vi "IV_ZAL_2015640414_P5.vi"(7 "Enum":T2(ring), 8 "error in":errorcluster, 10 "OPERADORES":T1={"Desplazamiento X"=0.0, "Desplazamiento Y"=500.0, "Giro"=0.0, "ZOOM"=0.0} {"ZOOM" min=0.1 max=10.0 step=0.01 scale=0.1..3.7; "Giro" scale=-360.0..360.0; "Desplazamiento Y" min=-500.0 max=500.0 step=1.0 scale=-200.0..200.0; "Desplazamiento X" min=-500.0 max=500.0 step=1.0 scale=-200.0..200.0}, 11 "IMAGEN 1":path) -> (0 "error out":errorcluster, 1 "HISTOGRAMA":dbl[][](graph), 2 "IMAGEN MODIFICADA":picture, 3 "IMAGEN ORIGINAL":picture)   [LabVIEW 2016]
doc: "SubVI para poder realizar distintas operaciones entre imagenes."
uses:
  <vilib>/imath/engines/lvmath2/RunTimeEngine/BuiltInFunctions/round/NIMS_round(DBL-S).vi
  <vilib>/imath/engines/lvmath2/RunTimeEngine/NodeEndStatement/NIMS_NodeEndStatement_Output.vi
  <instcachedir>/0/NIMS_NodeEndStatement_Output_53EC0D466D134D7ABD903AC30B43404B.lvgen/NIMS_NodeEndStatement_Output_53EC0D466D134D7ABD903AC30B43404B_010.vi
  <vilib>/imath/engines/lvmath2/RunTimeEngine/ErrorHandling/NIMS_Finalize Error.vi
  <instcachedir>/0/NIMS_NodeEndStatement_Output_53EC0D466D134D7ABD903AC30B43404B.lvgen/NIMS_NodeEndStatement_Output_53EC0D466D134D7ABD903AC30B43404B_001.vi
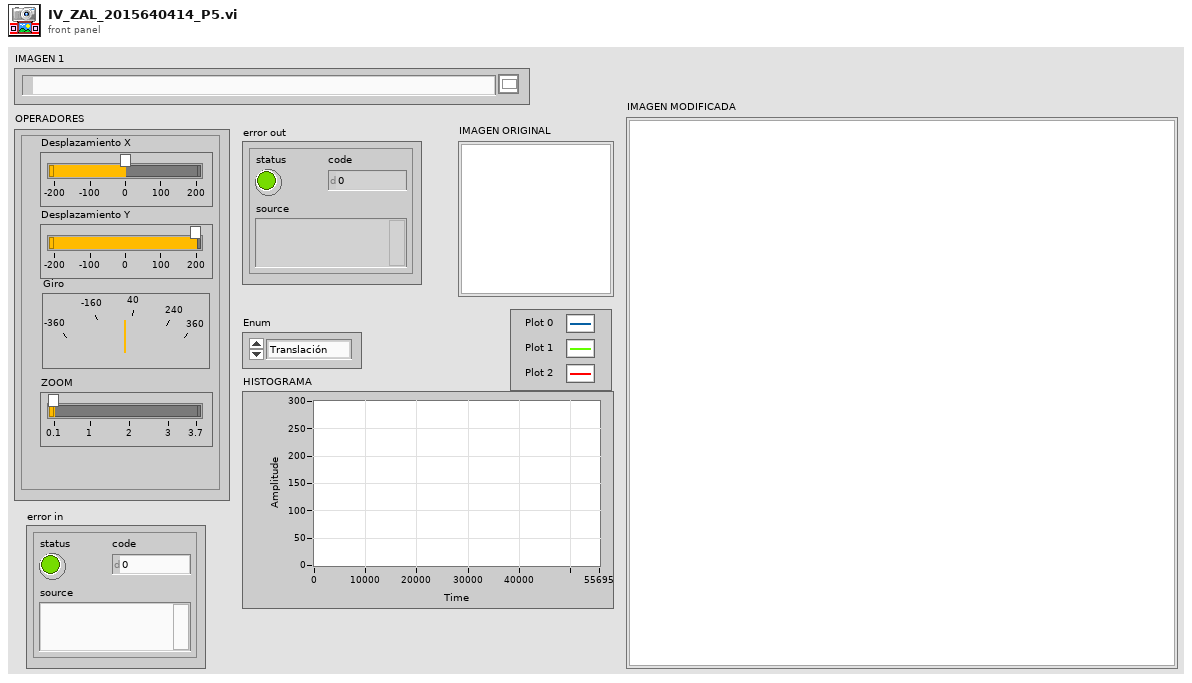
[diagram p1: front panel]
types:
  T1 = cluster{"Desplazamiento X":dbl, "Desplazamiento Y":dbl, "Giro":dbl, "ZOOM":dbl}
  T2 = enum16{"Translación", "Rotación", "Zoom", "GIROH", "GIROV", "Extracción", "Sustitución", "UNION"}
  T3 = typedef "imagedata.ctl" = cluster{"image type":i32, "image depth":i32, "image":u8[], "mask":u8[], "colors":u32[], "Rectangle":cluster{"left":i16, "top":i16, "right":i16, "bottom":i16}}
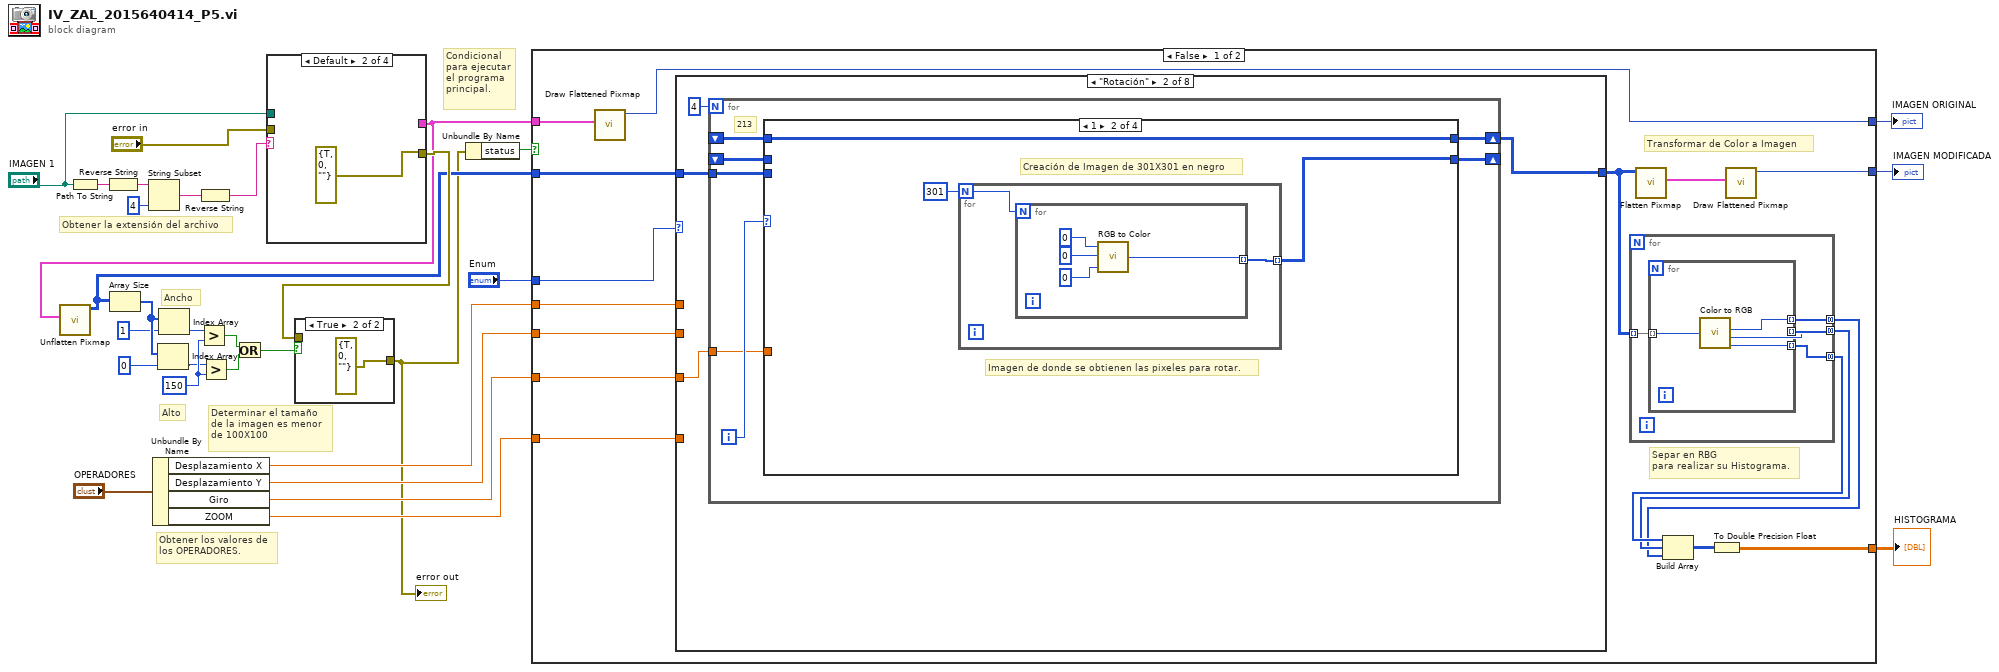
[diagram p0: block diagram]
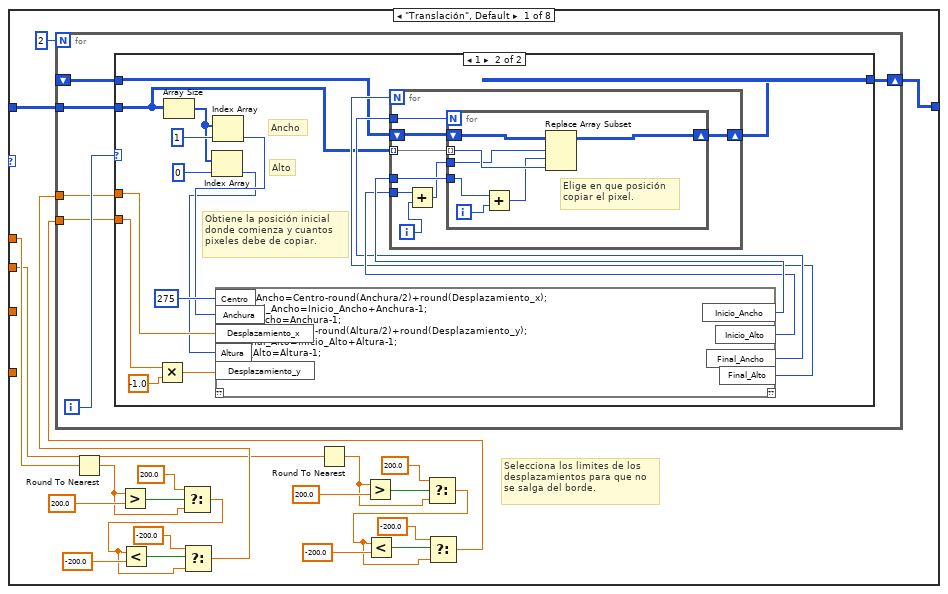
[diagram p3: hidden frame]
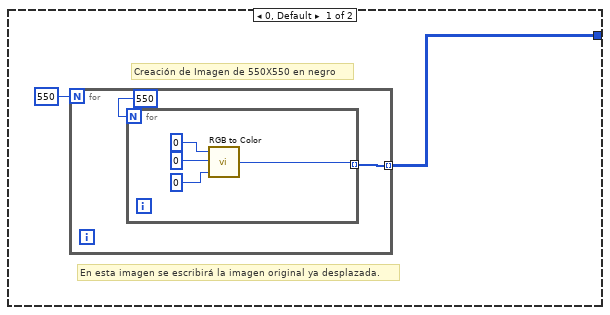
[diagram p4: hidden frame]
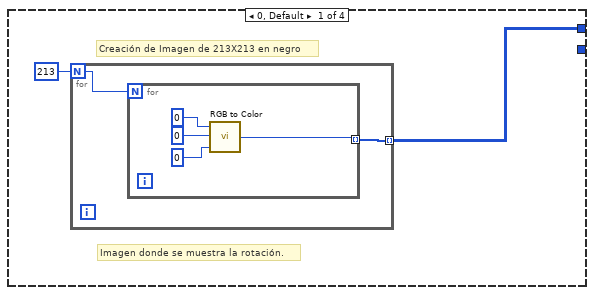
[diagram p5: hidden frame]
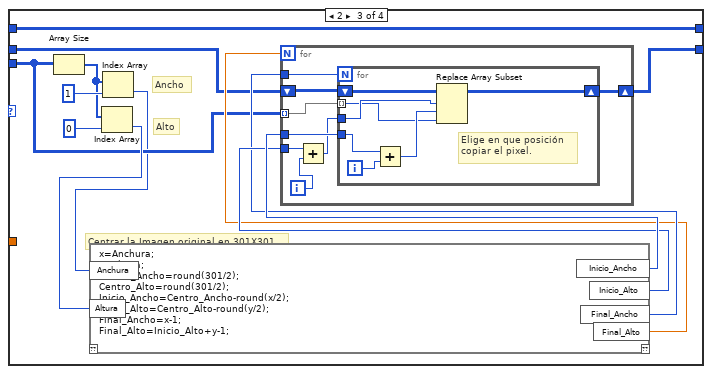
[diagram p6: hidden frame]
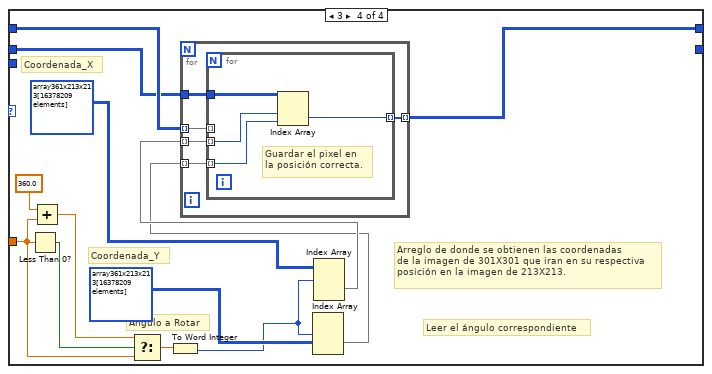
[diagram p7: hidden frame]
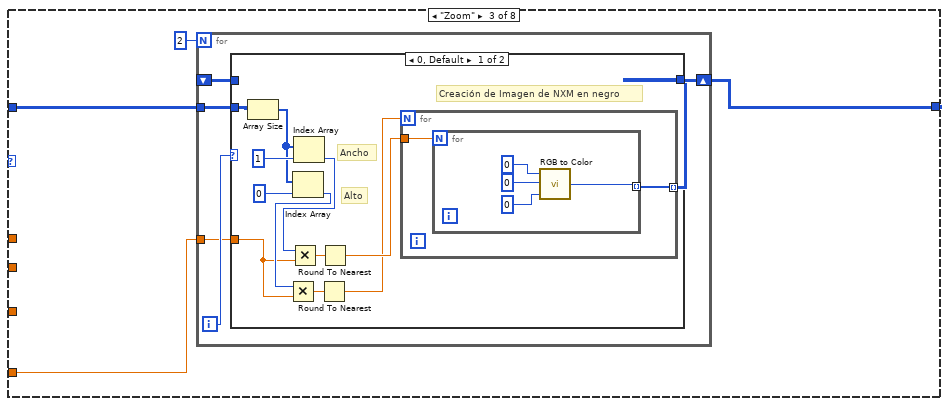
[diagram p8: hidden frame]
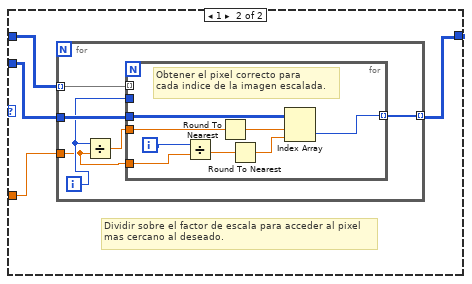
[diagram p9: hidden frame]
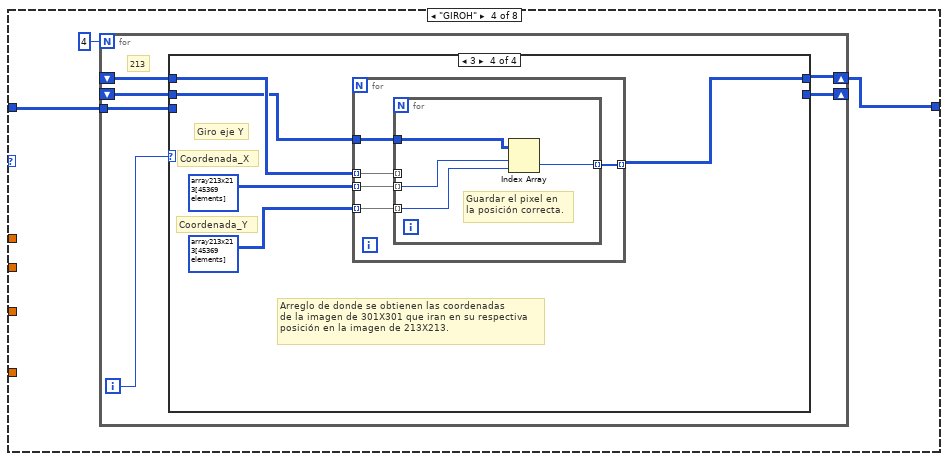
[diagram p10: hidden frame]
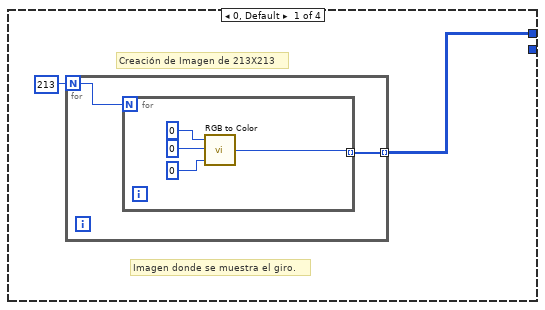
[diagram p11: hidden frame]
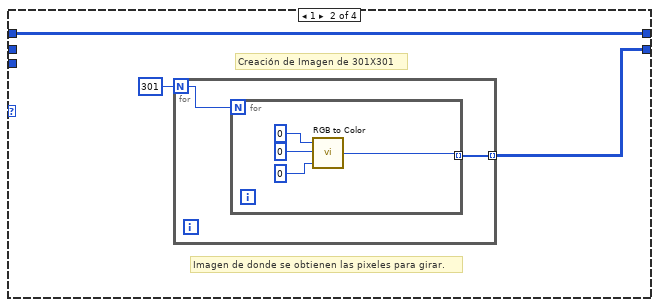
[diagram p12: hidden frame]
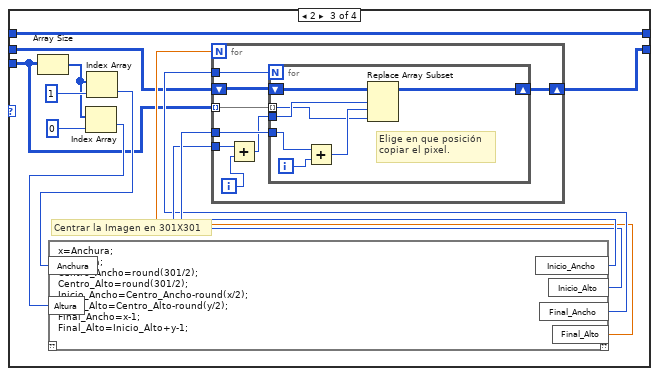
[diagram p13: hidden frame]
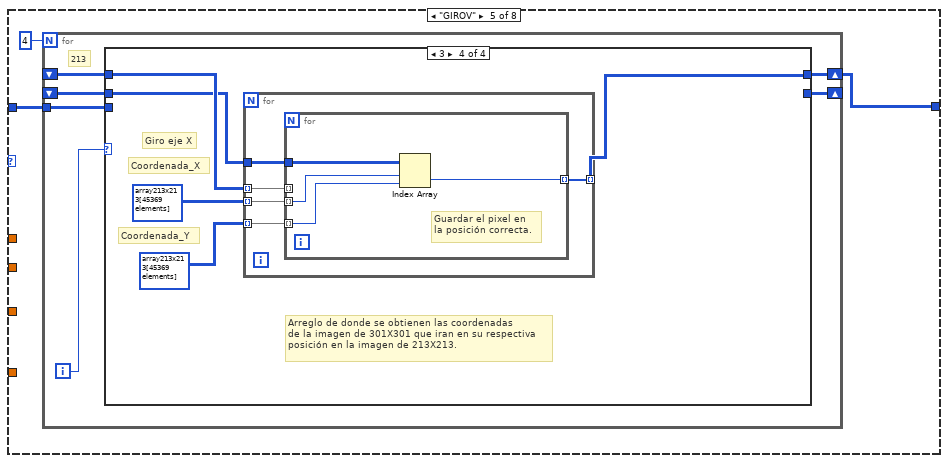
[diagram p14: hidden frame]
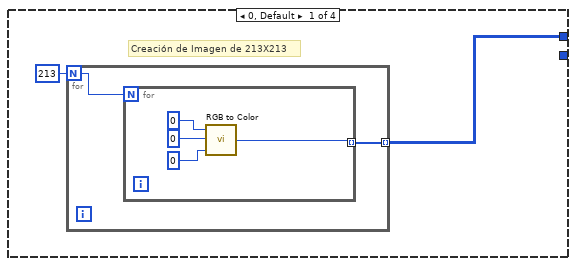
[diagram p15: hidden frame]
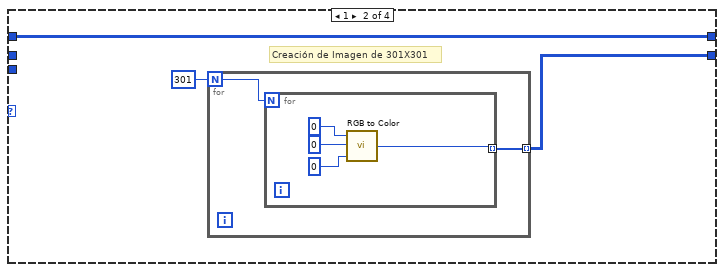
[diagram p16: hidden frame]
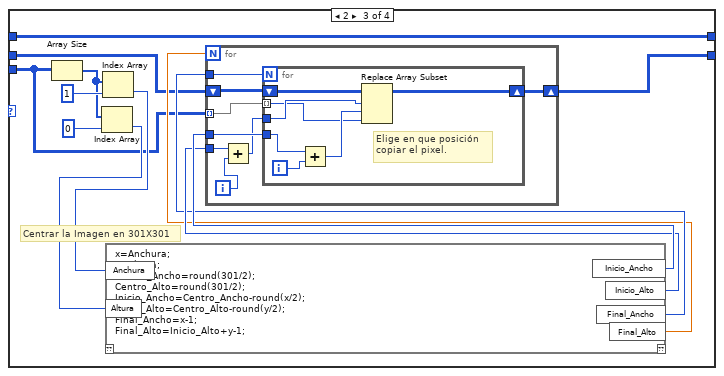
[diagram p17: hidden frame]
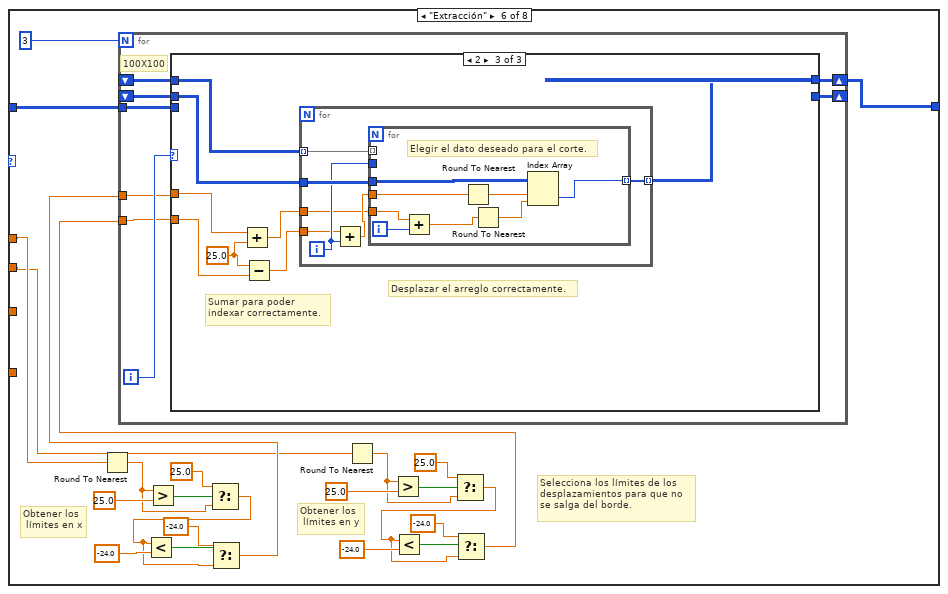
[diagram p18: hidden frame]
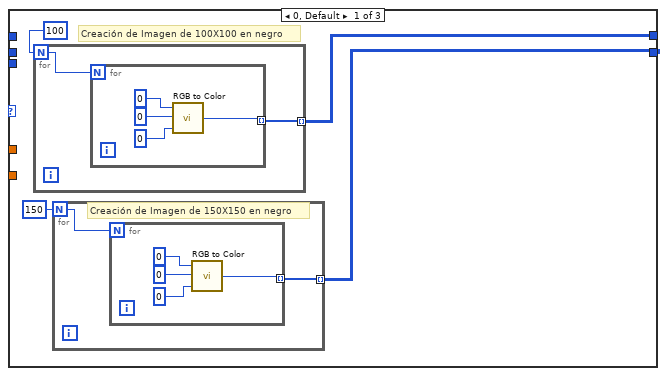
[diagram p19: hidden frame]
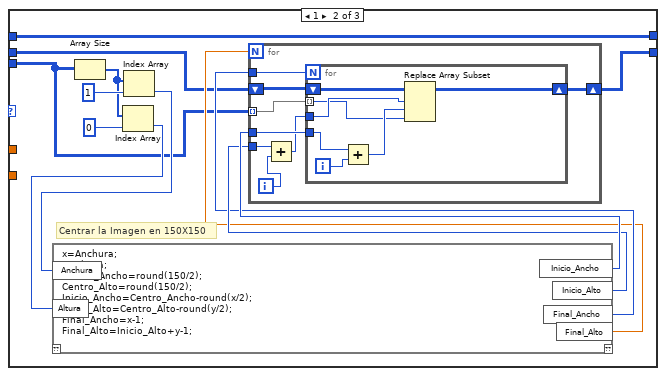
[diagram p20: hidden frame]
diagram:
  w18 = 150 ("y")
  # "Condicional\npara ejecutar\nel programa\nprincipal."
  # "Obtener los valores de\nlos OPERADORES."
  # "Determinar el tamaño\nde la imagen es menor\nde 100X100"
  # "Obtener la extensión del archivo"
  # "Alto"
  # "Ancho"
  n1 = Path To String(path="IMAGEN 1") -> (string=w1:string)
  n2 = Reverse String(1:w1) -> (0:w2:string)
  n3 = String Subset(string=w2, length (rest)=4 ("length (rest)")) -> (substring=w4:string)  [unwired: 1 in]
  n4 = Unbundle By Name("OPERADORES") -> ("Desplazamiento X"=w24:dbl, "Desplazamiento Y"=w25:dbl, "Giro"=w26:dbl, "ZOOM"=w27:dbl)
  n5 = Reverse String(1:w4) -> (0:w7:string)
  n6 = case shown="Default" w7 {
    tunnel: "IMAGEN 1" -> [w34 _ w39 w42]
    tunnel: "error in" -> [w33 _ w38 w41]
    tunnel: [w32 _ w37 w43] -> w20
    tunnel: [w31 errorcluster {"status"=TRUE, "code"=0, "source"=""} ("error in (no error)") w36 w40] -> w21
    frame ".JPEG", ".JPG", ".jpeg", ".jpg" {
      n7 = call <vilib>:"Read JPEG File.vi"("error in (no error)"=w33, "path to JPEG file"=w34) -> ("error out"=w31:errorcluster, "image data"=w32:T3)  [unwired: 7 in, 1 out]
    }
    frame Default {
    }
    frame ".PNG", ".png" {
      n8 = call <vilib>:"Read PNG File.vi"("error in (no error)"=w38, "path to PNG file"=w39) -> ("error out"=w36:errorcluster, "image data"=w37:T3)  [unwired: 7 in, 1 out]
    }
    frame ".BMP", ".bmp" {
      n9 = call <vilib>:"Read BMP File.vi"("error in (no error)"=w41, "path to BMP file"=w42) -> ("error out"=w40:errorcluster, "image data"=w43:T3)  [unwired: 7 in, 1 out]
    }
  }
  n10 = call <vilib>:"Unflatten Pixmap.vi"("image data"=w20) -> ("24-bit pixmap"=w19:u32[][])  [unwired: 4 in, 6 out]
  n11 = Array Size(array=w19) -> (size(s)=w12:i32[])
  n12 = Index Array(array=w12, index=0) -> (element=w14:i32)
  n13 = Index Array(array=w12, index=1) -> (element=w13:i32)
  n14 = Greater?(x=w13, y=w18) -> (0:w15:bool)
  n15 = Greater?(x=w14, y=w18) -> (0:w16:bool)
  n16 = Or(x=w15, y=w16) -> (x .or. y?=w22:bool)
  n17 = case shown="True" w22 {
    tunnel: [w44 errorcluster {"status"=TRUE, "code"=0, "source"=""} ("error in (no error)")] -> w17
    tunnel: w21 -> [w44 _]
    frame False {
    }
    frame True {
    }
  }
  "error out" <- w17
  n18 = Unbundle By Name(w17) -> ("status"=w8:bool)
  n19 = case shown="False" w8 {
    tunnel: w20 -> [w61 _]
    tunnel: "Enum" -> [w60 _]
    tunnel: w24 -> [w59 _]
    tunnel: w25 -> [w58 _]
    tunnel: w26 -> [w56 _]
    tunnel: w27 -> [w51 _]
    tunnel: w19 -> [w50 _]
    tunnel: [w48 _] -> w28
    tunnel: [w47 _] -> w29
    tunnel: [w46 _] -> w30
    frame False {
      # "Separ en RBG\npara realizar su Histograma."
      # "Transformar de Color a Imagen"
      n20 = call <vilib>:"Draw Flattened Pixmap.vi"("image data"=w61) -> ("new picture"=w46:picture)  [unwired: 8 in]
      n21 = case shown="\"Rotación\"" w60 {
        tunnel: w50 -> [w91 w207 w365 w411 w561 w713 w893 w1061]
        tunnel: w59 -> [w84 _ _ _ _ w712 w892 w1060]
        tunnel: w58 -> [w72 _ _ _ _ w711 w891 w1059]
        tunnel: [w70 w206 w367 w410 w560 w710 w890 w1058] -> w55
        tunnel: w56 -> [_ w205 _ _ _ _ _ _]
        tunnel: w51 -> [_ _ w366 _ _ _ _ _]
        frame "Translación", Default {
          # "Selecciona los limites de los\ndesplazamientos para que no\nse salga del borde."
          n22 = Round To Nearest(number=w84) -> (nearest integer value=w81:dbl)
          n23 = Greater?(x=w81, y=200.0) -> (0:w89:bool)
          n24 = Select(t=200.0, s=w89, f=w81) -> (s? t:f=w85:dbl)
          n25 = Less?(x=w85, y=-200.0) -> (x < y?=w90:bool)
          n26 = Select(t=-200.0, s=w90, f=w85) -> (s? t:f=w83:dbl)
          n27 = Round To Nearest(number=w72) -> (nearest integer value=w73:dbl)
          n28 = Greater?(x=w73, y=200.0) -> (0:w79:bool)
          n29 = Select(t=200.0, s=w79, f=w73) -> (s? t:f=w75:dbl)
          n30 = Less?(x=w75, y=-200.0) -> (x < y?=w80:bool)
          n31 = Select(t=-200.0, s=w80, f=w75) -> (s? t:f=w71:dbl)
          n32 = for {
            N: 2 -> [_]
            shift-right: [w97] -> w70
            shift-left: _ -> [w96]
            tunnel: w91 -> [w95]
            tunnel: w83 -> [w94]
            tunnel: w71 -> [w93]
            i -> [w98]
            n33 = case shown="1" w98 {
              tunnel: [w99 w110] -> w97
              tunnel: w96 -> [_ w111]
              tunnel: w95 -> [_ w112]
              tunnel: w94 -> [_ w120]
              tunnel: w93 -> [_ w109]
              frame 0, Default {
                # "En esta imagen se escribirá la imagen original ya desplazada."
                # "Creación de Imagen de 550X550 en negro"
                n34 = for {
                  N: 550 -> [_]
                  tunnel: [w101] -> w99 mode=indexing
                  n35 = for {
                    N: 550 -> [_]
                    tunnel: [w103] -> w101 mode=indexing
                    n36 = call <vilib>:"RGB to Color.vi"("B"=u8 0, "G"=u8 0, "R"=u8 0) -> ("Color"=w103:u32)
                  }
                }
              }
              frame 1 {
                # "Alto"
                # "Ancho"
                # "Obtiene la posición inicial\ndonde comienza y cuantos\npixeles debe de copiar."
                n37 = Multiply(x=w109, y=-1.0) -> (x*y=w107:dbl)
                n38 = Array Size(array=w112) -> (size(s)=w121:i32[])
                n39 = Index Array(array=w121, index=0) -> (element=w117:i32)
                n40 = Index Array(array=w121, index=1) -> (element=w118:i32)
                n41 = mathscript code="Inicio_Ancho=Centro-round(Anchura/2)+round(Desplazamiento_x);\n%%Final_Ancho=Inicio_Ancho+Anchura-1;\nFinal_Ancho=Anchura-1;\nInicio_Alto=Centro-round(Altura/2)+round(Desplazamiento_y);\n%%Final_Alto=Inicio_Alto+Altura-1;\nFinal_Alto=Altura-1;"("Centro"=275, "Anchura"=w118, "Desplazamiento_x"=w120, "Altura"=w117, "Desplazamiento_y"=w107) -> ("Inicio_Ancho"=w116:i32, "Inicio_Alto"=w115:i32, "Final_Ancho"=w114:i32, "Final_Alto"=w113:i32)  [unwired: 1 in, 1 out]
                n42 = for {
                  N: w113 -> [_]
                  tunnel: w116 -> [w130]
                  tunnel: w115 -> [w129]
                  tunnel: w114 -> [w127]
                  tunnel: w112 -> [w126] mode=indexing
                  shift-right: [w124] -> w110
                  shift-left: w111 -> [w125]
                  i -> [w131]
                  n43 = Add(x=w129, y=w131) -> (x+y=w128:i32)
                  n44 = for {
                    N: w127 -> [_]
                    tunnel: w130 -> [w137]
                    tunnel: w128 -> [w133]
                    tunnel: w126 -> [w134] mode=indexing
                    shift-right: [w135] -> w124
                    shift-left: w125 -> [w136]
                    i -> [w138]
                    # "Elige en que posición \ncopiar el pixel."
                    n45 = Add(x=w137, y=w138) -> (x+y=w132:i32)
                    n46 = Replace Array Subset(array=w136, new element=w134, index (row)=w133, index (col)=w132) -> (w135:u32[][])
                  }
                }
              }
            }
          }
        }
        frame "Rotación" {
          n47 = for {
            N: 4 -> [_]
            shift-right: [w213] -> w206
            shift-left: _ -> [w214]
            tunnel: w207 -> [w210]
            shift-right: [w212] -> _
            shift-left: _ -> [w211]
            tunnel: w205 -> [w209]
            i -> [w215]
            # "213"
            n48 = case shown="1" w215 {
              tunnel: [w216 w225 w236 w353] -> w213
              tunnel: w214 -> [_ w225 w236 w355]
              tunnel: [_ w224 w237 _] -> w212
              tunnel: w211 -> [_ _ w235 w354]
              tunnel: w210 -> [_ _ w234 _]
              tunnel: w209 -> [_ _ _ w348]
              frame 0, Default {
                # "Imagen donde se muestra la rotación."
                # "Creación de Imagen de 213X213 en negro"
                n49 = for {
                  N: 213 -> [w218]
                  tunnel: [w219] -> w216 mode=indexing
                  n50 = for {
                    N: w218 -> [_]
                    tunnel: [w220] -> w219 mode=indexing
                    n51 = call <vilib>:"RGB to Color.vi"("B"=u8 0, "G"=u8 0, "R"=u8 0) -> ("Color"=w220:u32)
                  }
                }
              }
              frame 1 {
                # "Imagen de donde se obtienen las pixeles para rotar."
                # "Creación de Imagen de 301X301 en negro"
                n52 = for {
                  N: 301 -> [w227]
                  tunnel: [w228] -> w224 mode=indexing
                  n53 = for {
                    N: w227 -> [_]
                    tunnel: [w229] -> w228 mode=indexing
                    n54 = call <vilib>:"RGB to Color.vi"("B"=u8 0, "G"=u8 0, "R"=u8 0) -> ("Color"=w229:u32)
                  }
                }
              }
              frame 2 {
                # "Alto"
                # "Ancho"
                # "Centrar la Imagen original en 301X301"
                n55 = Array Size(array=w234) -> (size(s)=w239:i32[])
                n56 = Index Array(array=w239, index=0) -> (element=w238:i32)
                n57 = Index Array(array=w239, index=1) -> (element=w233:i32)
                n58 = mathscript code="x=Anchura;\ny=Altura;\nCentro_Ancho=round(301/2);\nCentro_Alto=round(301/2);\nInicio_Ancho=Centro_Ancho-round(x/2);\nInicio_Alto=Centro_Alto-round(y/2);\nFinal_Ancho=x-1;\nFinal_Alto=Inicio_Alto+y-1;"("Anchura"=w233, "Altura"=w238) -> ("Inicio_Ancho"=w243:i32, "Inicio_Alto"=w242:i32, "Final_Ancho"=w241:i32, "Final_Alto"=w240:dbl)  [unwired: 1 in, 1 out]
                n59 = for {
                  N: w240 -> [_]
                  tunnel: w243 -> [w252]
                  tunnel: w242 -> [w251]
                  tunnel: w241 -> [w249]
                  shift-right: [w247] -> w237
                  shift-left: w235 -> [w248]
                  tunnel: w234 -> [w246] mode=indexing
                  i -> [w253]
                  n60 = Add(x=w251, y=w253) -> (x+y=w250:i32)
                  n61 = for {
                    N: w249 -> [_]
                    tunnel: w252 -> [w259]
                    tunnel: w250 -> [w257]
                    shift-right: [w258] -> w247
                    shift-left: w248 -> [w255]
                    tunnel: w246 -> [w254] mode=indexing
                    i -> [w260]
                    # "Elige en que posición \ncopiar el pixel."
                    n62 = Add(x=w259, y=w260) -> (x+y=w256:i32)
                    n63 = Replace Array Subset(array=w255, new element=w254, index (row)=w257, index (col)=w256) -> (w258:u32[][])
                  }
                }
              }
              frame 3 {
                # "Leer el ángulo correspondiente"
                # "Arreglo de donde se obtienen las coordenadas\nde la imagen de 301X301 que iran en su respectiva\nposición en la imagen de 213X213."
                # "Ángulo a Rotar"
                # "Coordenada_X"
                # "Coordenada_Y"
                n64 = Less Than 0?(x=w348) -> (x < 0?=w349:bool)
                n65 = Add(x=360.0, y=w348) -> (x+y=w346:dbl)
                n66 = Select(t=w346, s=w349, f=w348) -> (s? t:f=w345:dbl)
                n67 = To Word Integer(number=w345) -> (16bit integer=w343:i16)
                n68 = Index Array(array=i16[][][] array361x213x213[16378209 elements] ("Coordenada_y"), index (dim 0)=w343) -> (element=w350:i16[][])  [unwired: 2 in]
                n69 = Index Array(array=i16[][][] array361x213x213[16378209 elements] ("Coordenada_x"), index (dim 0)=w343) -> (element=w351:i16[][])  [unwired: 2 in]
                n70 = for {
                  tunnel: w355 -> [w360] mode=indexing
                  tunnel: w351 -> [w359] mode=indexing
                  tunnel: w350 -> [w358] mode=indexing
                  tunnel: w354 -> [w357]
                  tunnel: [w356] -> w353 mode=indexing
                  n71 = for {
                    tunnel: w360 -> [_] mode=indexing
                    tunnel: w359 -> [w363] mode=indexing
                    tunnel: w358 -> [w362] mode=indexing
                    tunnel: w357 -> [w364]
                    tunnel: [w361] -> w356 mode=indexing
                    # "Guardar el pixel en\nla posición correcta."
                    n72 = Index Array(array=w364, index (row)=w363, index (col)=w362) -> (element=w361:u32)
                  }
                }
              }
            }
          }
        }
        frame "Zoom" {
          n73 = for {
            N: 2 -> [_]
            shift-right: [w372] -> w367
            shift-left: _ -> [w371]
            tunnel: w365 -> [w370]
            tunnel: w366 -> [w369]
            i -> [w373]
            n74 = case shown="0, Default" w373 {
              tunnel: [w385 w392] -> w372
              tunnel: w371 -> [_ w395]
              tunnel: w370 -> [w381 w394]
              tunnel: w369 -> [w376 w393]
              frame 0, Default {
                # "Alto"
                # "Ancho"
                # "Creación de Imagen de NXM en negro"
                n75 = Array Size(array=w381) -> (size(s)=w382:i32[])
                n76 = Index Array(array=w382, index=0) -> (element=w377:i32)
                n77 = Multiply(x=w377, y=w376) -> (x*y=w379:dbl)
                n78 = Index Array(array=w382, index=1) -> (element=w378:i32)
                n79 = Multiply(x=w378, y=w376) -> (x*y=w380:dbl)
                n80 = Round To Nearest(number=w379) -> (nearest integer value=w374:dbl)
                n81 = Round To Nearest(number=w380) -> (nearest integer value=w375:dbl)
                n82 = for {
                  N: w374 -> [_]
                  tunnel: [w387] -> w385 mode=indexing
                  tunnel: w375 -> [w386]
                  n83 = for {
                    N: w386 -> [_]
                    tunnel: [w388] -> w387 mode=indexing
                    n84 = call <vilib>:"RGB to Color.vi"("B"=u8 0, "G"=u8 0, "R"=u8 0) -> ("Color"=w388:u32)
                  }
                }
              }
              frame 1 {
                # "Dividir sobre el factor de escala para acceder al pixel\nmas cercano al deseado."
                n85 = for {
                  tunnel: w395 -> [w401] mode=indexing
                  tunnel: w394 -> [w400]
                  tunnel: w393 -> [w396]
                  tunnel: [w397] -> w392 mode=indexing
                  i -> [w399]
                  n86 = Divide(x=w399, y=w396) -> (x/y=w398:dbl)
                  n87 = for {
                    tunnel: w399 -> [_]
                    tunnel: w401 -> [_] mode=indexing
                    tunnel: w400 -> [w409]
                    tunnel: w398 -> [w404]
                    tunnel: [w403] -> w397 mode=indexing
                    tunnel: w396 -> [w402]
                    i -> [w405]
                    # "Obtener el pixel correcto para\ncada indice de la imagen escalada."
                    n88 = Divide(x=w405, y=w402) -> (x/y=w406:dbl)
                    n89 = Round To Nearest(number=w404) -> (nearest integer value=w408:dbl)
                    n90 = Round To Nearest(number=w406) -> (nearest integer value=w407:dbl)
                    n91 = Index Array(array=w409, index (row)=w408, index (col)=w407) -> (element=w403:u32)
                  }
                }
              }
            }
          }
        }
        frame "GIROH" {
          n92 = for {
            N: 4 -> [_]
            shift-right: [w416] -> w410
            shift-left: _ -> [w417]
            tunnel: w411 -> [w413]
            shift-right: [w415] -> _
            shift-left: _ -> [w414]
            i -> [w418]
            # "213"
            n93 = case shown="3" w418 {
              tunnel: [w419 w428 w438 w548] -> w416
              tunnel: w417 -> [_ w428 w438 w550]
              tunnel: [_ w427 w439 _] -> w415
              tunnel: w414 -> [_ _ w437 w549]
              tunnel: w413 -> [_ _ w436 _]
              frame 0, Default {
                # "Imagen donde se muestra el giro."
                # "Creación de Imagen de 213X213"
                n94 = for {
                  N: 213 -> [w421]
                  tunnel: [w422] -> w419 mode=indexing
                  n95 = for {
                    N: w421 -> [_]
                    tunnel: [w423] -> w422 mode=indexing
                    n96 = call <vilib>:"RGB to Color.vi"("B"=u8 0, "G"=u8 0, "R"=u8 0) -> ("Color"=w423:u32)
                  }
                }
              }
              frame 1 {
                # "Imagen de donde se obtienen las pixeles para girar."
                # "Creación de Imagen de 301X301"
                n97 = for {
                  N: 301 -> [w430]
                  tunnel: [w431] -> w427 mode=indexing
                  n98 = for {
                    N: w430 -> [_]
                    tunnel: [w432] -> w431 mode=indexing
                    n99 = call <vilib>:"RGB to Color.vi"("B"=u8 0, "G"=u8 0, "R"=u8 0) -> ("Color"=w432:u32)
                  }
                }
              }
              frame 2 {
                # "Centrar la Imagen en 301X301"
                n100 = Array Size(array=w436) -> (size(s)=w442:i32[])
                n101 = Index Array(array=w442, index=0) -> (element=w440:i32)
                n102 = Index Array(array=w442, index=1) -> (element=w441:i32)
                n103 = mathscript code="x=Anchura;\ny=Altura;\nCentro_Ancho=round(301/2);\nCentro_Alto=round(301/2);\nInicio_Ancho=Centro_Ancho-round(x/2);\nInicio_Alto=Centro_Alto-round(y/2);\nFinal_Ancho=x-1;\nFinal_Alto=Inicio_Alto+y-1;"("Anchura"=w441, "Altura"=w440) -> ("Inicio_Ancho"=w446:i32, "Inicio_Alto"=w445:i32, "Final_Ancho"=w444:i32, "Final_Alto"=w443:dbl)  [unwired: 1 in, 1 out]
                n104 = for {
                  N: w443 -> [_]
                  tunnel: w446 -> [w455]
                  tunnel: w445 -> [w454]
                  tunnel: w444 -> [w452]
                  shift-right: [w450] -> w439
                  shift-left: w437 -> [w451]
                  tunnel: w436 -> [w449] mode=indexing
                  i -> [w456]
                  n105 = Add(x=w454, y=w456) -> (x+y=w453:i32)
                  n106 = for {
                    N: w452 -> [_]
                    tunnel: w455 -> [w462]
                    tunnel: w453 -> [w460]
                    shift-right: [w461] -> w450
                    shift-left: w451 -> [w458]
                    tunnel: w449 -> [w457] mode=indexing
                    i -> [w463]
                    # "Elige en que posición \ncopiar el pixel."
                    n107 = Add(x=w462, y=w463) -> (x+y=w459:i32)
                    n108 = Replace Array Subset(array=w458, new element=w457, index (row)=w460, index (col)=w459) -> (w461:u32[][])
                  }
                }
              }
              frame 3 {
                # "Arreglo de donde se obtienen las coordenadas\nde la imagen de 301X301 que iran en su respectiva\nposición en la imagen de 213X213."
                # "Giro eje Y"
                # "Coordenada_Y"
                # "Coordenada_X"
                n109 = for {
                  tunnel: w550 -> [w555] mode=indexing
                  tunnel: i16[][] array213x213[45369 elements] ("Coordenada_x") -> [w554] mode=indexing
                  tunnel: i16[][] array213x213[45369 elements] ("Coordenada_y") -> [w553] mode=indexing
                  tunnel: w549 -> [w552]
                  tunnel: [w551] -> w548 mode=indexing
                  n110 = for {
                    tunnel: w555 -> [_] mode=indexing
                    tunnel: w554 -> [w558] mode=indexing
                    tunnel: w553 -> [w557] mode=indexing
                    tunnel: w552 -> [w559]
                    tunnel: [w556] -> w551 mode=indexing
                    # "Guardar el pixel en\nla posición correcta."
                    n111 = Index Array(array=w559, index (row)=w558, index (col)=w557) -> (element=w556:u32)
                  }
                }
              }
            }
          }
        }
        frame "GIROV" {
          n112 = for {
            N: 4 -> [_]
            shift-right: [w566] -> w560
            shift-left: _ -> [w567]
            tunnel: w561 -> [w563]
            shift-right: [w565] -> _
            shift-left: _ -> [w564]
            i -> [w568]
            # "213"
            n113 = case shown="3" w568 {
              tunnel: [w569 w578 w588 w698] -> w566
              tunnel: w567 -> [_ w578 w588 w700]
              tunnel: [_ w577 w589 _] -> w565
              tunnel: w564 -> [_ _ w587 w699]
              tunnel: w563 -> [_ _ w586 _]
              frame 0, Default {
                # "Creación de Imagen de 213X213"
                n114 = for {
                  N: 213 -> [w571]
                  tunnel: [w572] -> w569 mode=indexing
                  n115 = for {
                    N: w571 -> [_]
                    tunnel: [w573] -> w572 mode=indexing
                    n116 = call <vilib>:"RGB to Color.vi"("B"=u8 0, "G"=u8 0, "R"=u8 0) -> ("Color"=w573:u32)
                  }
                }
              }
              frame 1 {
                # "Creación de Imagen de 301X301"
                n117 = for {
                  N: 301 -> [w580]
                  tunnel: [w581] -> w577 mode=indexing
                  n118 = for {
                    N: w580 -> [_]
                    tunnel: [w582] -> w581 mode=indexing
                    n119 = call <vilib>:"RGB to Color.vi"("B"=u8 0, "G"=u8 0, "R"=u8 0) -> ("Color"=w582:u32)
                  }
                }
              }
              frame 2 {
                # "Centrar la Imagen en 301X301"
                n120 = Array Size(array=w586) -> (size(s)=w592:i32[])
                n121 = Index Array(array=w592, index=0) -> (element=w590:i32)
                n122 = Index Array(array=w592, index=1) -> (element=w591:i32)
                n123 = mathscript code="x=Anchura;\ny=Altura;\nCentro_Ancho=round(301/2);\nCentro_Alto=round(301/2);\nInicio_Ancho=Centro_Ancho-round(x/2);\nInicio_Alto=Centro_Alto-round(y/2);\nFinal_Ancho=x-1;\nFinal_Alto=Inicio_Alto+y-1;"("Anchura"=w591, "Altura"=w590) -> ("Inicio_Ancho"=w596:i32, "Inicio_Alto"=w595:i32, "Final_Ancho"=w594:i32, "Final_Alto"=w593:dbl)  [unwired: 1 in, 1 out]
                n124 = for {
                  N: w593 -> [_]
                  tunnel: w596 -> [w605]
                  tunnel: w595 -> [w604]
                  tunnel: w594 -> [w602]
                  shift-right: [w600] -> w589
                  shift-left: w587 -> [w601]
                  tunnel: w586 -> [w599] mode=indexing
                  i -> [w606]
                  n125 = Add(x=w604, y=w606) -> (x+y=w603:i32)
                  n126 = for {
                    N: w602 -> [_]
                    tunnel: w605 -> [w612]
                    tunnel: w603 -> [w610]
                    shift-right: [w611] -> w600
                    shift-left: w601 -> [w608]
                    tunnel: w599 -> [w607] mode=indexing
                    i -> [w613]
                    # "Elige en que posición \ncopiar el pixel."
                    n127 = Add(x=w612, y=w613) -> (x+y=w609:i32)
                    n128 = Replace Array Subset(array=w608, new element=w607, index (row)=w610, index (col)=w609) -> (w611:u32[][])
                  }
                }
              }
              frame 3 {
                # "Arreglo de donde se obtienen las coordenadas\nde la imagen de 301X301 que iran en su respectiva\nposición en la imagen de 213X213."
                # "Giro eje X"
                # "Coordenada_X"
                # "Coordenada_Y"
                n129 = for {
                  tunnel: w700 -> [w705] mode=indexing
                  tunnel: i16[][] array213x213[45369 elements] ("Coordenada_x") -> [w704] mode=indexing
                  tunnel: i16[][] array213x213[45369 elements] ("Coordenada_y") -> [w703] mode=indexing
                  tunnel: w699 -> [w702]
                  tunnel: [w701] -> w698 mode=indexing
                  n130 = for {
                    tunnel: w705 -> [_] mode=indexing
                    tunnel: w704 -> [w708] mode=indexing
                    tunnel: w703 -> [w707] mode=indexing
                    tunnel: w702 -> [w709]
                    tunnel: [w706] -> w701 mode=indexing
                    # "Guardar el pixel en\nla posición correcta."
                    n131 = Index Array(array=w709, index (row)=w708, index (col)=w707) -> (element=w706:u32)
                  }
                }
              }
            }
          }
        }
        frame "Extracción" {
          # "Selecciona los límites de los\ndesplazamientos para que no\nse salga del borde."
          # "Obtener los\n límites en y"
          # "Obtener los\n límites en x"
          n132 = Round To Nearest(number=w712) -> (nearest integer value=w723:dbl)
          n133 = Greater?(x=w723, y=25.0) -> (0:w730:bool)
          n134 = Select(t=25.0, s=w730, f=w723) -> (s? t:f=w726:dbl)
          n135 = Less?(x=w726, y=-24.0) -> (x < y?=w731:bool)
          n136 = Select(t=-24.0, s=w731, f=w726) -> (s? t:f=w725:dbl)
          n137 = Round To Nearest(number=w711) -> (nearest integer value=w715:dbl)
          n138 = Greater?(x=w715, y=25.0) -> (0:w721:bool)
          n139 = Select(t=25.0, s=w721, f=w715) -> (s? t:f=w717:dbl)
          n140 = Less?(x=w717, y=-24.0) -> (x < y?=w722:bool)
          n141 = Select(t=-24.0, s=w722, f=w717) -> (s? t:f=w714:dbl)
          n142 = for {
            N: 3 -> [_]
            shift-right: [w739] -> w710
            shift-left: _ -> [w738]
            tunnel: w713 -> [w737]
            tunnel: w725 -> [w736]
            tunnel: w714 -> [w735]
            shift-right: [w734] -> _
            shift-left: _ -> [w733]
            i -> [w740]
            # "100X100"
            n143 = case shown="2" w740 {
              tunnel: [w743 w757 w873] -> w739
              tunnel: w738 -> [_ w757 w874]
              tunnel: w737 -> [_ w760 _]
              tunnel: w736 -> [_ _ w871]
              tunnel: w735 -> [_ _ w867]
              tunnel: [w741 w759 _] -> w734
              tunnel: w733 -> [_ w758 w872]
              frame 0, Default {
                # "Creación de Imagen de 100X100 en negro"
                n144 = for {
                  N: 100 -> [w751]
                  tunnel: [w752] -> w743 mode=indexing
                  n145 = for {
                    N: w751 -> [_]
                    tunnel: [w753] -> w752 mode=indexing
                    n146 = call <vilib>:"RGB to Color.vi"("B"=u8 0, "G"=u8 0, "R"=u8 0) -> ("Color"=w753:u32)
                  }
                }
                n147 = for {
                  N: 150 -> [w745]
                  tunnel: [w746] -> w741 mode=indexing
                  # "Creación de Imagen de 150X150 en negro"
                  n148 = for {
                    N: w745 -> [_]
                    tunnel: [w747] -> w746 mode=indexing
                    n149 = call <vilib>:"RGB to Color.vi"("B"=u8 0, "G"=u8 0, "R"=u8 0) -> ("Color"=w747:u32)
                  }
                }
              }
              frame 1 {
                # "Centrar la Imagen en 150X150"
                n150 = Array Size(array=w760) -> (size(s)=w763:i32[])
                n151 = Index Array(array=w763, index=0) -> (element=w761:i32)
                n152 = Index Array(array=w763, index=1) -> (element=w762:i32)
                n153 = mathscript code="x=Anchura;\ny=Altura;\nCentro_Ancho=round(150/2);\nCentro_Alto=round(150/2);\nInicio_Ancho=Centro_Ancho-round(x/2);\nInicio_Alto=Centro_Alto-round(y/2);\nFinal_Ancho=x-1;\nFinal_Alto=Inicio_Alto+y-1;"("Anchura"=w762, "Altura"=w761) -> ("Inicio_Ancho"=w767:i32, "Inicio_Alto"=w766:i32, "Final_Ancho"=w765:i32, "Final_Alto"=w764:dbl)  [unwired: 1 in, 1 out]
                n154 = for {
                  N: w764 -> [_]
                  tunnel: w767 -> [w776]
                  tunnel: w766 -> [w775]
                  tunnel: w765 -> [w773]
                  shift-right: [w771] -> w759
                  shift-left: w758 -> [w772]
                  tunnel: w760 -> [w770] mode=indexing
                  i -> [w777]
                  n155 = Add(x=w775, y=w777) -> (x+y=w774:i32)
                  n156 = for {
                    N: w773 -> [_]
                    tunnel: w776 -> [w783]
                    tunnel: w774 -> [w781]
                    shift-right: [w782] -> w771
                    shift-left: w772 -> [w779]
                    tunnel: w770 -> [w778] mode=indexing
                    i -> [w784]
                    n157 = Add(x=w783, y=w784) -> (x+y=w780:i32)
                    n158 = Replace Array Subset(array=w779, new element=w778, index (row)=w781, index (col)=w780) -> (w782:u32[][])
                  }
                }
              }
              frame 2 {
                w868 = 25.0 ("y")
                # "Desplazar el arreglo correctamente."
                # "Sumar para poder \nindexar correctamente."
                n159 = Add(x=w871, y=w868) -> (x+y=w869:dbl)
                n160 = Subtract(x=w868, y=w867) -> (x-y=w870:dbl)
                n161 = for {
                  tunnel: w874 -> [w881] mode=indexing
                  tunnel: w872 -> [w880]
                  tunnel: [w879] -> w873 mode=indexing
                  tunnel: w870 -> [w876]
                  tunnel: w869 -> [w875]
                  i -> [w878]
                  n162 = Add(x=w876, y=w878) -> (x+y=w877:dbl)
                  n163 = for {
                    tunnel: w878 -> [_]
                    tunnel: w881 -> [_] mode=indexing
                    tunnel: w880 -> [w889]
                    tunnel: [w886] -> w879 mode=indexing
                    tunnel: w877 -> [w884]
                    tunnel: w875 -> [w882]
                    i -> [w885]
                    # "Elegir el dato deseado para el corte."
                    n164 = Add(x=w882, y=w885) -> (x+y=w883:dbl)
                    n165 = Round To Nearest(number=w884) -> (nearest integer value=w888:dbl)
                    n166 = Round To Nearest(number=w883) -> (nearest integer value=w887:dbl)
                    n167 = Index Array(array=w889, index (row)=w888, index (col)=w887) -> (element=w886:u32)
                  }
                }
              }
            }
          }
        }
        frame "Sustitución" {
          # "Selecciona los límites de los\ndesplazamientos para que no\nse salga del borde."
          # "Obtener los límites en y"
          # "Obtener los límites en x"
          n168 = Round To Nearest(number=w892) -> (nearest integer value=w903:dbl)
          n169 = Greater?(x=w903, y=25.0) -> (0:w910:bool)
          n170 = Select(t=25.0, s=w910, f=w903) -> (s? t:f=w906:dbl)
          n171 = Less?(x=w906, y=-24.0) -> (x < y?=w911:bool)
          n172 = Select(t=-24.0, s=w911, f=w906) -> (s? t:f=w905:dbl)
          n173 = Round To Nearest(number=w891) -> (nearest integer value=w895:dbl)
          n174 = Greater?(x=w895, y=25.0) -> (0:w901:bool)
          n175 = Select(t=25.0, s=w901, f=w895) -> (s? t:f=w897:dbl)
          n176 = Less?(x=w897, y=-24.0) -> (x < y?=w902:bool)
          n177 = Select(t=-24.0, s=w902, f=w897) -> (s? t:f=w894:dbl)
          n178 = for {
            N: 3 -> [_]
            shift-right: [w917] -> w890
            shift-left: _ -> [w916]
            tunnel: w893 -> [w915]
            tunnel: w905 -> [w914]
            tunnel: w894 -> [w913]
            i -> [w918]
            # "150X150"
            n179 = case shown="2" w918 {
              tunnel: [w919 w927 w1040] -> w917
              tunnel: w916 -> [_ w928 w1043]
              tunnel: w915 -> [_ w929 _]
              tunnel: w914 -> [_ _ w1042]
              tunnel: w913 -> [_ _ w1036]
              frame 0, Default {
                # "Creación de Imagen de 150X150 en negro"
                n180 = for {
                  N: 150 -> [w921]
                  tunnel: [w922] -> w919 mode=indexing
                  n181 = for {
                    N: w921 -> [_]
                    tunnel: [w923] -> w922 mode=indexing
                    n182 = call <vilib>:"RGB to Color.vi"("B"=u8 0, "G"=u8 0, "R"=u8 0) -> ("Color"=w923:u32)
                  }
                }
              }
              frame 1 {
                # "Centrar la Imagen en 150X150"
                n183 = Array Size(array=w929) -> (size(s)=w932:i32[])
                n184 = Index Array(array=w932, index=0) -> (element=w930:i32)
                n185 = Index Array(array=w932, index=1) -> (element=w931:i32)
                n186 = mathscript code="x=Anchura;\ny=Altura;\nCentro_Ancho=round(150/2);\nCentro_Alto=round(150/2);\nInicio_Ancho=Centro_Ancho-round(x/2);\nInicio_Alto=Centro_Alto-round(y/2);\nFinal_Ancho=x-1;\nFinal_Alto=Inicio_Alto+y-1;"("Anchura"=w931, "Altura"=w930) -> ("Inicio_Ancho"=w936:i32, "Inicio_Alto"=w935:i32, "Final_Ancho"=w934:i32, "Final_Alto"=w933:dbl)  [unwired: 1 in, 1 out]
                n187 = for {
                  N: w933 -> [_]
                  tunnel: w936 -> [w945]
                  tunnel: w935 -> [w944]
                  tunnel: w934 -> [w942]
                  shift-right: [w940] -> w927
                  shift-left: w928 -> [w941]
                  tunnel: w929 -> [w939] mode=indexing
                  i -> [w946]
                  n188 = Add(x=w944, y=w946) -> (x+y=w943:i32)
                  n189 = for {
                    N: w942 -> [_]
                    tunnel: w945 -> [w952]
                    tunnel: w943 -> [w950]
                    shift-right: [w951] -> w940
                    shift-left: w941 -> [w948]
                    tunnel: w939 -> [w947] mode=indexing
                    i -> [w953]
                    # "Guardar el pixel en\nla posición correcta."
                    n190 = Add(x=w952, y=w953) -> (x+y=w949:i32)
                    n191 = Replace Array Subset(array=w948, new element=w947, index (row)=w950, index (col)=w949) -> (w951:u32[][])
                  }
                }
              }
              frame 2 {
                w1041 = u32[][] array100x100[10000 elements]  # Imagen 100X100
                w1037 = 25.0 ("y")
                # "Sumar para poder indexar desde cero."
                n192 = Subtract(x=w1037, y=w1036) -> (x-y=w1039:dbl)
                n193 = Add(x=w1042, y=w1037) -> (x+y=w1038:dbl)
                n194 = for {
                  tunnel: w1039 -> [w1047]
                  tunnel: w1038 -> [w1046]
                  tunnel: w1041 -> [w1045] mode=indexing
                  shift-right: [w1044] -> w1040
                  shift-left: w1043 -> [w1050]
                  i -> [w1049]
                  n195 = Add(x=w1047, y=w1049) -> (x+y=w1048:dbl)
                  n196 = for {
                    tunnel: w1049 -> [_]
                    tunnel: w1048 -> [w1051]
                    tunnel: w1046 -> [w1056]
                    tunnel: w1045 -> [w1054] mode=indexing
                    shift-right: [w1053] -> w1044
                    shift-left: w1050 -> [w1055]
                    i -> [w1057]
                    # "Escoger los puntos a Sustituir."
                    n197 = Add(x=w1056, y=w1057) -> (x+y=w1052:dbl)
                    n198 = Replace Array Subset(array=w1055, new element=w1054, index (row)=w1051, index (col)=w1052) -> (w1053:u32[][])
                  }
                }
              }
            }
          }
        }
        frame "UNION" {
          # "Selecciona los límites de los\ndesplazamientos para que no\nse salga del borde."
          # "Obtener los\n límites en y"
          # "Obtener los\n límites en x"
          n199 = Round To Nearest(number=w1060) -> (nearest integer value=w1071:dbl)
          n200 = Greater?(x=w1071, y=25.0) -> (0:w1078:bool)
          n201 = Select(t=25.0, s=w1078, f=w1071) -> (s? t:f=w1074:dbl)
          n202 = Less?(x=w1074, y=-24.0) -> (x < y?=w1079:bool)
          n203 = Select(t=-24.0, s=w1079, f=w1074) -> (s? t:f=w1073:dbl)
          n204 = Round To Nearest(number=w1059) -> (nearest integer value=w1063:dbl)
          n205 = Greater?(x=w1063, y=25.0) -> (0:w1069:bool)
          n206 = Select(t=25.0, s=w1069, f=w1063) -> (s? t:f=w1065:dbl)
          n207 = Less?(x=w1065, y=-24.0) -> (x < y?=w1070:bool)
          n208 = Select(t=-24.0, s=w1070, f=w1065) -> (s? t:f=w1062:dbl)
          n209 = for {
            N: 3 -> [_]
            shift-right: [w1087] -> w1058
            shift-left: _ -> [w1086]
            tunnel: w1061 -> [w1085]
            tunnel: w1073 -> [w1084]
            tunnel: w1062 -> [w1083]
            shift-right: [w1082] -> _
            shift-left: _ -> [w1081]
            i -> [w1088]
            # "100X100"
            n210 = case shown="2" w1088 {
              tunnel: [w1089 w1113 w1227] -> w1087
              tunnel: w1086 -> [_ w1113 w1228]
              tunnel: w1085 -> [_ w1116 _]
              tunnel: w1084 -> [_ _ w1233]
              tunnel: w1083 -> [_ _ w1224]
              tunnel: [w1098 w1115 _] -> w1082
              tunnel: w1081 -> [_ w1114 w1234]
              frame 0, Default {
                w1090 = u32[][] array100x100[10000 elements]  # Vegeta 100X100
                w1097 = u32[][] array100x100[10000 elements]  # Goku 100X100
                # "Cargar la segunda imagen\ndesde 100 a 300."
                # "Cargar la primera\nimagen en desde 1\na 100."
                # "Creación de Imagen de 300X100 en negro"
                n211 = for {
                  N: 100 -> [_]
                  tunnel: [w1108] -> w1096 mode=indexing
                  n212 = for {
                    N: 300 -> [_]
                    tunnel: [w1109] -> w1108 mode=indexing
                    n213 = call <vilib>:"RGB to Color.vi"("B"=u8 0, "G"=u8 0, "R"=u8 0) -> ("Color"=w1109:u32)
                  }
                }
                n214 = for {
                  N: 150 -> [w1101]
                  tunnel: [w1102] -> w1098 mode=indexing
                  # "Creación de Imagen de 150X150 en negro"
                  n215 = for {
                    N: w1101 -> [_]
                    tunnel: [w1103] -> w1102 mode=indexing
                    n216 = call <vilib>:"RGB to Color.vi"("B"=u8 0, "G"=u8 0, "R"=u8 0) -> ("Color"=w1103:u32)
                  }
                }
                n217 = Replace Array Subset(array=w1096, new element=w1097, index (row)=0, index (col)=0 ("disabled index (col)")) -> (w1093:u32[][])
                n218 = Replace Array Subset(array=w1093, new element=w1090, index (row)=0 ("disabled index (row)"), index (col)=199 ("disabled index (col)")) -> (w1089:u32[][])
              }
              frame 1 {
                # "Centrar la Imagen en 150X150"
                n219 = Array Size(array=w1116) -> (size(s)=w1119:i32[])
                n220 = Index Array(array=w1119, index=0) -> (element=w1117:i32)
                n221 = Index Array(array=w1119, index=1) -> (element=w1118:i32)
                n222 = mathscript code="x=Anchura;\ny=Altura;\nCentro_Ancho=round(150/2);\nCentro_Alto=round(150/2);\nInicio_Ancho=Centro_Ancho-round(x/2);\nInicio_Alto=Centro_Alto-round(y/2);\nFinal_Ancho=x-1;\nFinal_Alto=Inicio_Alto+y-1;"("Anchura"=w1118, "Altura"=w1117) -> ("Inicio_Ancho"=w1123:i32, "Inicio_Alto"=w1122:i32, "Final_Ancho"=w1121:i32, "Final_Alto"=w1120:dbl)  [unwired: 1 in, 1 out]
                n223 = for {
                  N: w1120 -> [_]
                  tunnel: w1123 -> [w1132]
                  tunnel: w1122 -> [w1131]
                  tunnel: w1121 -> [w1129]
                  shift-right: [w1127] -> w1115
                  shift-left: w1114 -> [w1128]
                  tunnel: w1116 -> [w1126] mode=indexing
                  i -> [w1133]
                  n224 = Add(x=w1131, y=w1133) -> (x+y=w1130:i32)
                  n225 = for {
                    N: w1129 -> [_]
                    tunnel: w1132 -> [w1139]
                    tunnel: w1130 -> [w1137]
                    shift-right: [w1138] -> w1127
                    shift-left: w1128 -> [w1135]
                    tunnel: w1126 -> [w1134] mode=indexing
                    i -> [w1140]
                    n226 = Add(x=w1139, y=w1140) -> (x+y=w1136:i32)
                    n227 = Replace Array Subset(array=w1135, new element=w1134, index (row)=w1137, index (col)=w1136) -> (w1138:u32[][])
                  }
                }
              }
              frame 2 {
                w1223 = 25.0 ("y")
                # "Colocar en nuevo\narreglo de la posición\n100 a 200."
                # "Sumar para poder\n indexar desde correctamente."
                n228 = Add(x=w1233, y=w1223) -> (x+y=w1226:dbl)
                n229 = Subtract(x=w1223, y=w1224) -> (x-y=w1225:dbl)
                n230 = for {
                  N: 100 -> [w1235]
                  tunnel: w1234 -> [w1241]
                  tunnel: [w1240] -> w1229 mode=indexing
                  tunnel: w1225 -> [w1237]
                  tunnel: w1226 -> [w1236]
                  i -> [w1239]
                  n231 = Add(x=w1237, y=w1239) -> (x+y=w1238:dbl)
                  n232 = for {
                    N: w1235 -> [_]
                    tunnel: w1239 -> [_]
                    tunnel: w1241 -> [w1249]
                    tunnel: [w1248] -> w1240 mode=indexing
                    tunnel: w1238 -> [w1246]
                    tunnel: w1236 -> [w1244]
                    i -> [w1247]
                    # "Elegir el dato deseado para el corte."
                    n233 = Add(x=w1244, y=w1247) -> (x+y=w1245:dbl)
                    n234 = Round To Nearest(number=w1246) -> (nearest integer value=w1243:dbl)
                    n235 = Round To Nearest(number=w1245) -> (nearest integer value=w1242:dbl)
                    n236 = Index Array(array=w1249, index (row)=w1243, index (col)=w1242) -> (element=w1248:u32)
                  }
                }
                n237 = Replace Array Subset(array=w1228, new element=w1229, index (row)=0 ("disabled index (row)"), index (col)=99 ("disabled index (col)")) -> (w1227:u32[][])
              }
            }
          }
        }
      }
      n238 = for {
        tunnel: w55 -> [w65] mode=indexing
        tunnel: [w64] -> w53 mode=concatenating
        tunnel: [w63] -> w54 mode=concatenating
        tunnel: [w62] -> w52 mode=concatenating
        n239 = for {
          tunnel: w65 -> [w69] mode=indexing
          tunnel: [w67] -> w64 mode=indexing
          tunnel: [w68] -> w63 mode=indexing
          tunnel: [w66] -> w62 mode=indexing
          n240 = call <vilib>:"Color to RGB.vi"("Color"=w69) -> ("R"=w66:u8, "G"=w67:u8, "B"=w68:u8)  [unwired: 1 out]
        }
      }
      n241 = call <vilib>:"Flatten Pixmap.vi"("24-bit pixmap"=w55) -> ("image data"=w57:T3)  [unwired: 10 in]
      n242 = Build Array(w54, w53, w52) -> (w49:u8[][])
      n243 = To Double Precision Float(number=w49) -> (double precision float=w47:dbl[][])
      n244 = call <vilib>:"Draw Flattened Pixmap.vi"("image data"=w57) -> ("new picture"=w48:picture)  [unwired: 8 in]
    }
    frame True {
      # "Si es incorrecto el archivo no ejecuta nada."
    }
  }
  "IMAGEN MODIFICADA" <- w28
  "HISTOGRAMA" <- w29
  "IMAGEN ORIGINAL" <- w30
